vi "PF_cutAndBin.vi"(0 "Filename for atoms":path=path "c:/data/tempfiles/redPAS10VODT100msinter200mshold28080.000msh200000usd4.600dac20atoms.bny", 1 "Buffer address":i32=164036608, 3 "File Path for \nbackground image":path=path "c:/data/tempfiles/redPAS10VODT100msinter200mshold28080.000msh200000usd4.600dac20back.bny", 5 "Input Array":dbl[][](array[numeric])=array1024x1280[1310720 elements], 7 "error in":errorcluster={"status"=FALSE, "code"=0, "source"="Start camera.vi: No error - function call successful"}, 8 "boardid":i32, 9 "x bin":dbl=1.0, 11 "Continuous scan?\n(images not saved)":bool, 13 "DoubleShutter?":bool, 16 "# of images to sum":i32=6, 21 "Buffer number":i32, 24 "Size":i32=2621440) -> (17 "saved image dimensions":i32[](array[numeric])=[1024, 1280], 20 "Atoms Graph":dbl[][](graph), 23 "Background image":dbl[][](graph), 25 "Uncut Image":dbl[][](graph), 27 "error out":errorcluster={"status"=FALSE, "code"=0, "source"="Get buffer status.vi: No error - function call successful"})   [LabVIEW 2015]
uses:
  <vilib>/Utility/file.llb/Write To Spreadsheet File (DBL).vi
panel:
  in  "Save as Binary?":bool=TRUE
  out "bg avg":ext format="%.2f"
  out "Numeric":i32=2
  out "Atoms - Background":dbl[][](graph)
  out "Atoms Average":ext=651.4701080322266 format="%.2f"
  out "Average of Atoms minus Background":ext=651.4701080322266 format="%.2f"
  # "This is hard-wired.  No path is \npassed from the outside."
  # "x bin"
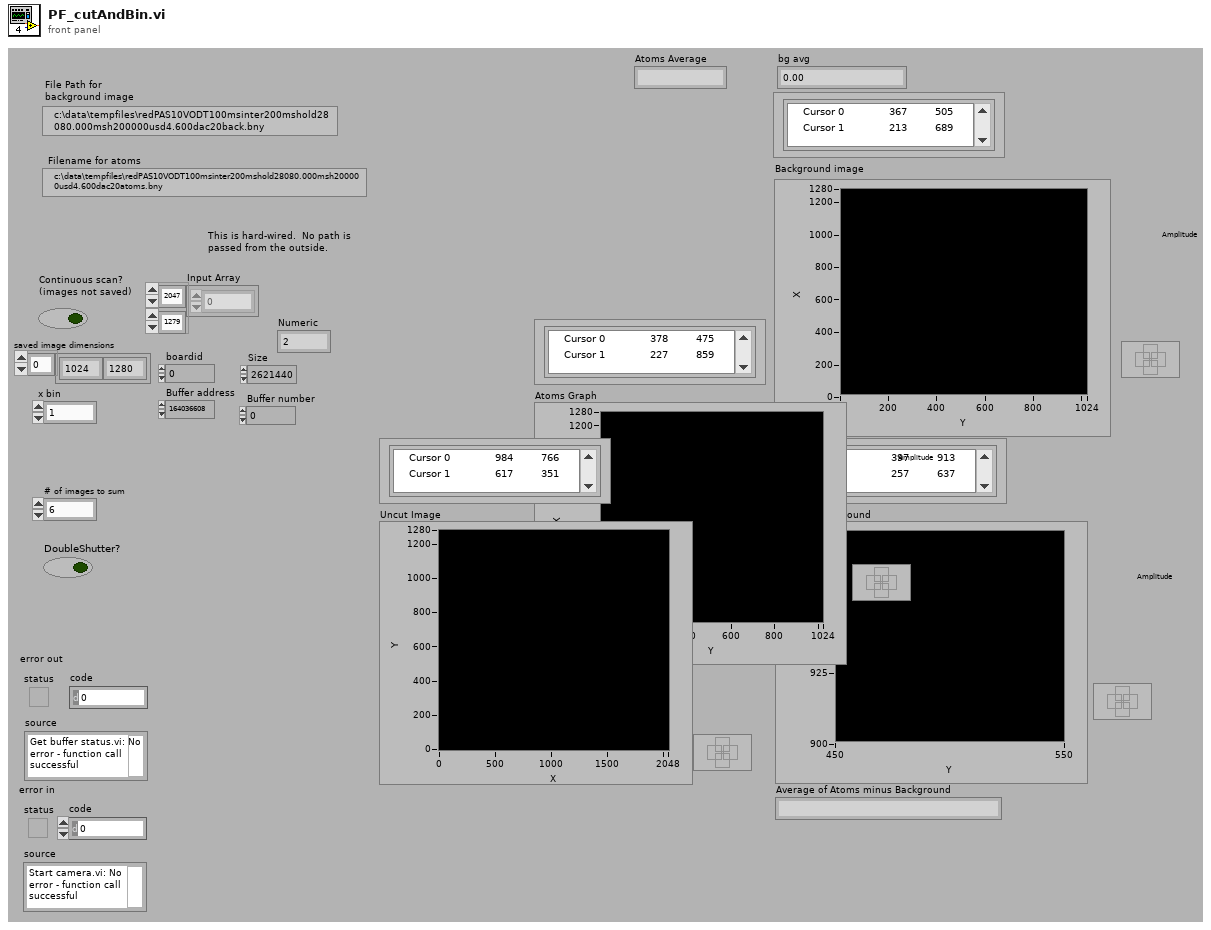
[diagram p1: front panel]
types:
  T1 = cluster{"Write":bool, "Write done":bool, "Queued":bool, "Cancelled":bool, "Select":bool, "Select done":bool, "Burst":bool, "Size":bool, "Event":bool, "Timeout":bool, "Open":i32, "Map":i32, "Exposure":i32[], "Offset":i32[], "Size":i32[], "Transfer":i32[], "Total Size":i32}
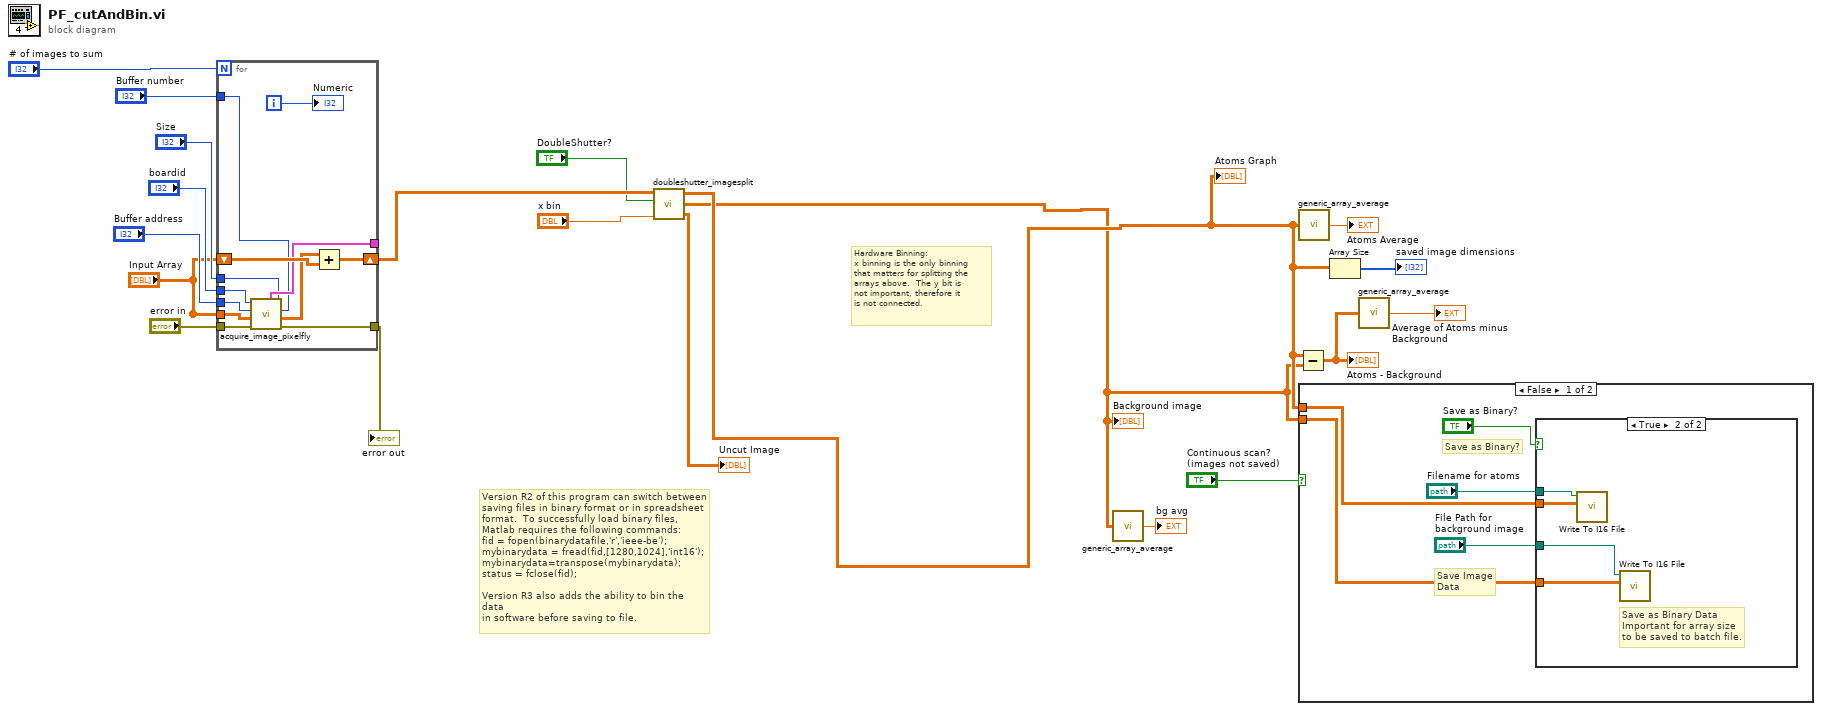
[diagram p0: block diagram]
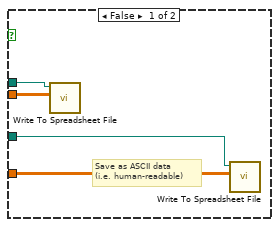
[diagram p2: hidden frame]
diagram:
  # "Version R2 of this program can switch between\nsaving files in binary format or in spreadsheet\nformat.  To successfully load binary files,\nMatlab requires the following commands:\nfid = fopen(binarydatafile,'r','ieee-be');\nmybinarydata = fread(fid,[1280,1024],'int16');\nmybinarydata=transpose(mybinarydata);\nstatus = fclose(fid);\n\nVersion R3 also adds the ability to bin the data\nin software before saving to file."
  # "Hardware Binning:\nx binning is the only binning\nthat matters for splitting the\narrays above.  The y bit is\nnot important, therefore it\nis not connected."
  n1 = for {
    N: "# of images to sum" -> [_]
    shift-right: [w29] -> w8
    shift-left: "Input Array" -> [w31]
    tunnel: [w32] -> w19
    tunnel: "error in" -> [w30]
    tunnel: "Input Array" -> [w27]
    tunnel: "boardid" -> [w25]
    tunnel: "Buffer address" -> [w24]
    tunnel: [w23] -> _
    tunnel: "Buffer number" -> [w22]
    tunnel: "Size" -> [w21]
    i -> [w26]
    n2 = call "acquire_image_pixelfly.vi"("boardid"=w25, "Buffer address"=w24, "Array input"=w27, "error in"=w30, "Size"=w21, "Buffer number"=w22) -> ("Buffer status"=w23:T1, "image array"=w28:dbl[][], "error out"=w32:errorcluster)
    n3 = Add(x=w28, y=w31) -> (x+y=w29:dbl[][])
    "Numeric" <- w26
  }
  "error out" <- w19
  n4 = call "doubleshutter_imagesplit.vi"("image array"=w8, "DoubleShutter?"="DoubleShutter?", "x bin"="x bin") -> ("lower half - atoms"=w2:dbl[][], "upper half - background"=w1:dbl[][], "Uncut Image"=→"Uncut Image":dbl[][])  [unwired: 2 in]
  "Atoms Graph" <- w2
  "Background image" <- w1
  n5 = call "generic_array_average.vi"("Array int 32"=w1) -> ("Average"=→"bg avg":ext)
  n6 = Subtract(x=w2, y=w1) -> (x-y=w12:dbl[][])
  "Atoms - Background" <- w12
  n7 = call "generic_array_average.vi"("Array int 32"=w2) -> ("Average"=→"Atoms Average":ext)
  n8 = case shown="False" "Continuous scan?\n(images not saved)" {
    tunnel: w2 -> [w34 _]
    tunnel: w1 -> [w33 _]
    frame False {
      # "Save as Binary?"
      # "Save Image\nData"
      n9 = case shown="True" "Save as Binary?" {
        tunnel: "File Path for \nbackground image" -> [w41 w43]
        tunnel: "Filename for atoms" -> [w40 w45]
        tunnel: w34 -> [w39 w44]
        tunnel: w33 -> [w38 w42]
        frame False {
          # "Save as ASCII data\n(i.e. human-readable)"
          n10 = call-poly <vilib>:"Write To Spreadsheet File.vi"("2D data"=w39, "file path (dialog if empty)"=w40) -> ()  [unwired: 6 in, 1 out]
          n11 = call-poly <vilib>:"Write To Spreadsheet File.vi"("2D data"=w38, "file path (dialog if empty)"=w41) -> ()  [unwired: 6 in, 1 out]
        }
        frame True {
          # "Save as Binary Data\nImportant for array size\nto be saved to batch file."
          n12 = call <vilib>:"Write To I16 File.vi"("2D array"=w44, "file path (dialog if empty)"=w45) -> ()  [unwired: 5 in, 1 out]
          n13 = call <vilib>:"Write To I16 File.vi"("2D array"=w42, "file path (dialog if empty)"=w43) -> ()  [unwired: 5 in, 1 out]
        }
      }
    }
    frame True {
      # "Don't save images\nwhen continuous."
    }
  }
  n14 = Array Size(array=w2) -> (size(s)=→"saved image dimensions":i32[])
  n15 = call "generic_array_average.vi"("Array int 32"=w12) -> ("Average"=→"Average of Atoms minus Background":ext)
